vi "CRYO_MASTER_temp_0911.vi"() -> ()   [LabVIEW 2017] (continued)
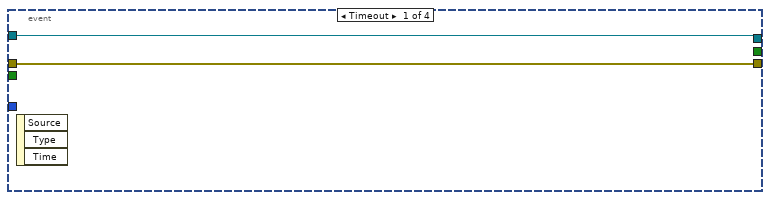
[diagram p3: hidden frame]
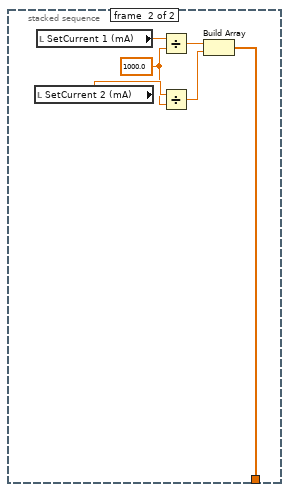
[diagram p8: hidden frame]
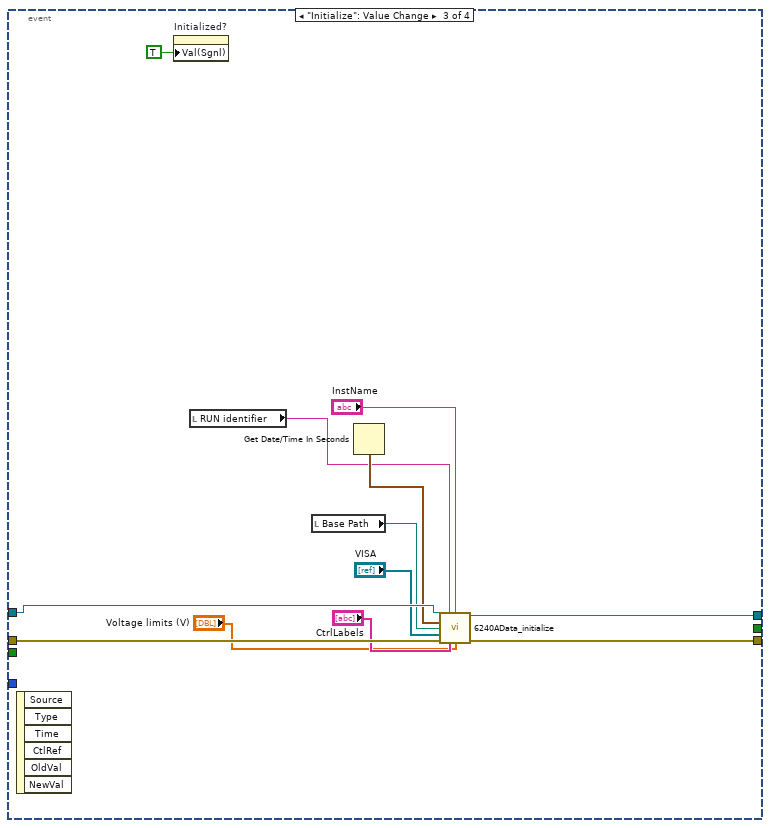
[diagram p10: hidden frame]
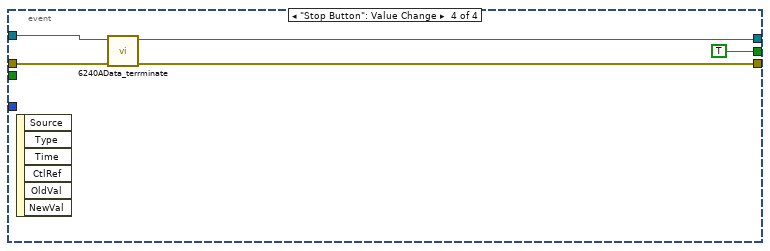
[diagram p11: hidden frame]
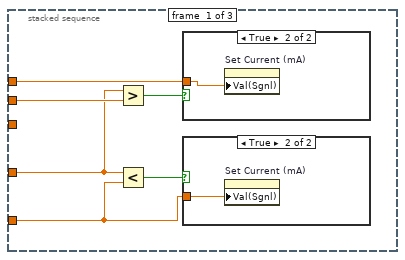
[diagram p12: hidden frame]
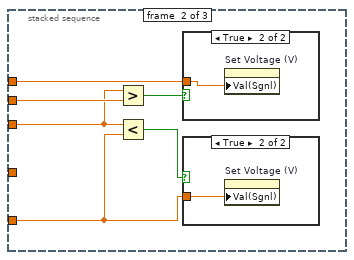
[diagram p15: hidden frame]
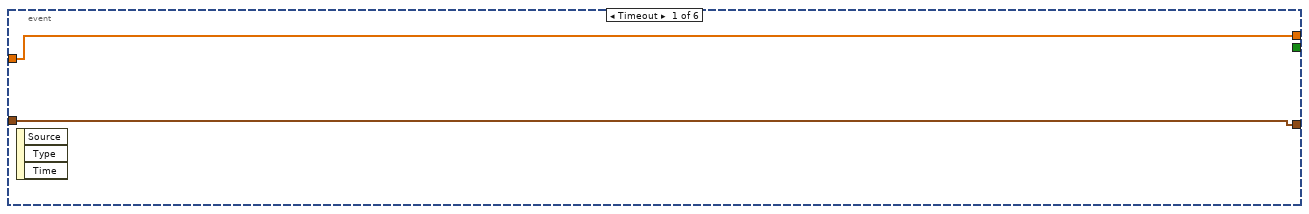
[diagram p18: hidden frame]
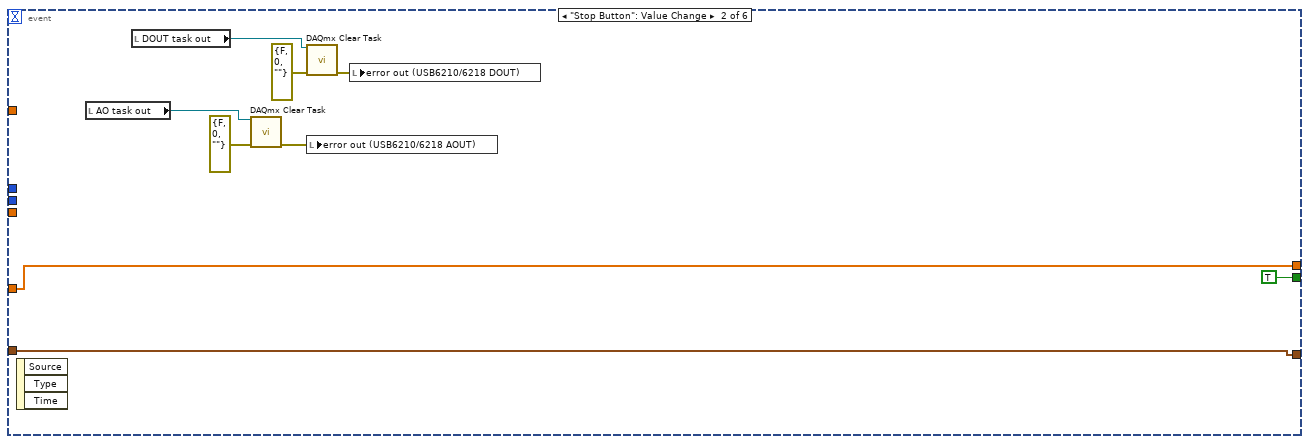
[diagram p19: hidden frame]
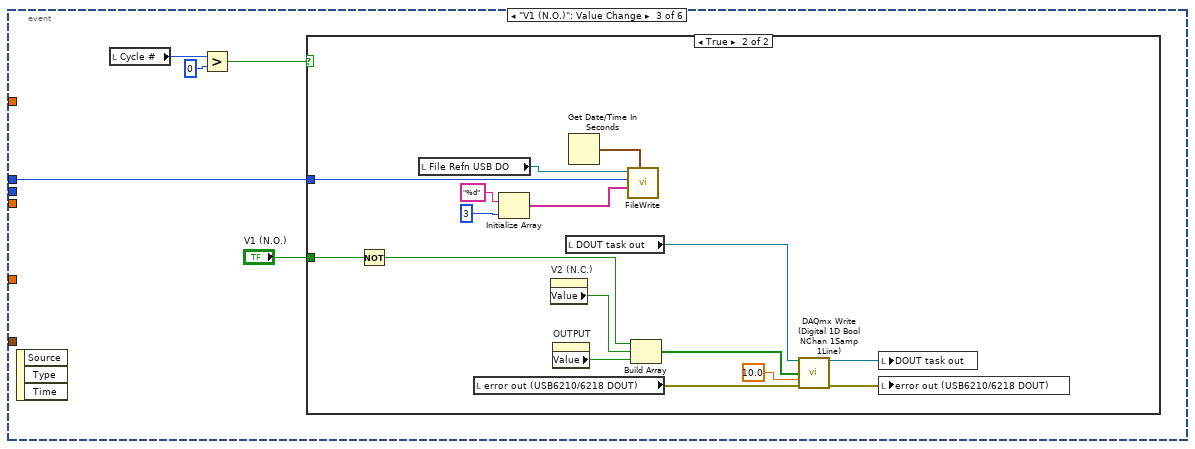
[diagram p20: hidden frame]
        "Time of Last Measurement (USB6218)" <- w698
        "Last Vol \n(USB6218)" <- w685
        n285 = call-dynamic "USBData_convert.vi"("Save every ... measurements"=w679, "MeasurementIndex"=w680, "error in (no error)"=w697, "LastDataAcquired"=w685, "TimeMeasuremeent"=w698, "USBData in"=w701) -> ("error out"=w696:errorcluster, "LeakDet_FULL"=w691:dbl, "LastDataConverted"=w686:dbl[], "USBData out"=w694:refnum<class "USBData.lvclass">)  [unwired: 2 in]
        n286 = call "USBData_read.vi"("USBData in"=w694, "error in (no error)"=w696) -> ("Status"=w687:T5, "USBData out"=w693:refnum<class "USBData.lvclass">, "Data"=w692:T15, "Basic"=w684:T16, "error out"=w695:errorcluster)  [unwired: 2 in, 2 out]
        n287 = local write "USB6218 Status"(w687) -> ()
        n288 = Unbundle By Name(w684) -> ("ReadLeakDet?"=w690:bool)
        n289 = Unbundle By Name(w684) -> ("Labels"=w683:string[])
        n290 = case shown="True" w690 {
          tunnel: w686 -> [w702 w705]
          tunnel: w691 -> [_ w704]
          tunnel: [w702 w703] -> w689
          frame False {
          }
          frame True {
            n291 = Build Array (concatenate)(w705, w704) -> (w703:dbl[])
          }
        }
        "Last Data \n(USB6218)" <- w689
      }
      frame True {
        n292 = Get Date/Time In Seconds() -> (seconds since 1Jan1904=w715:timestamp)
        n293 = call-dynamic "USBData_initialize.vi"("USBData in"=w711, "SeriesSetting"="USB6218 Config", "BasePath"=w710, "RunName"=w709, "FileName"="InstName (USB6218)", "error in (no error)"=w708, "RUN start time"=w715) -> ("Status"=w706:T5, "USBData out"=w724:refnum<class "USBData.lvclass">, "error out"=w725:errorcluster)  [unwired: 4 in, 2 out]
        n294 = local write "USB6218 Status"(w706) -> ()
        n295 = call "USBData_read.vi"("USBData in"=w724, "error in (no error)"=w725) -> ("Status"=w714:T5, "USBData out"=w721:refnum<class "USBData.lvclass">, "Data"=w722:T15, "Basic"=w716:T16, "error out"=w723:errorcluster)  [unwired: 2 in, 2 out]
        n296 = local write "USB6218 Status"(w714) -> ()
        n297 = Unbundle By Name(w716) -> ("ReadLeakDet?"=w720:bool, "Labels"=w713:string[])
        n298 = Array Size(array=w713) -> (size(s)=w719:i32)
        n299 = case shown="True" w720 {
          tunnel: w719 -> [w726 w728]
          tunnel: [w726 w727] -> w717
          frame False {
          }
          frame True {
            n300 = Add(x=w728, y=1) -> (x+y=w727:i32)
          }
        }
        n301 = Initialize Array(TRUE ("Activate 2"), w717) -> ()  [unwired: 1 out]
      }
    }
    "error out (USB6218)" <- w414
    n302 = case shown="False" w411 {
      tunnel: [w1080 w1095] -> w453
      tunnel: [w1075 w1094] -> w472
      tunnel: [w1078 w1093] -> w454
      tunnel: w422 -> [w1079 _]
      tunnel: w471 -> [w1069 w1088]
      tunnel: w470 -> [w1070 w1087]
      tunnel: w410 -> [_ w1086]
      tunnel: w409 -> [_ w1085]
      tunnel: [w1067 timestamp[] [] ("TimeArray")] -> w469
      tunnel: [w1066 dbl[][] [] ("DataArray")] -> w468
      frame False {
        w1073 = 24 ("index")
        n303 = local read "Record interval"() -> (w1064:i64)
        n304 = call-dynamic "LSI218Data_measure.vi"("LSI218Data in"=w1070, "MeasurementIndex"=w1079, "error in (no error)"=w1069, "save every ... measurements"=w1064) -> ("TimeMeasuremeent"=→"Time of Last Measurement (LSI218)":timestamp, "Active?"=w1074:bool[], "LSI218Data out"=w1078:refnum<class "LSI218Data.lvclass">, "LastMeasurementConfig"=→"LastMeasurementConfig (218)":T11, "LastData"=w1068:dbl[], "Status"=w1075:u16, "TimeArray"=w1067:timestamp[], "DataArray"=w1066:dbl[][], "error out"=w1080:errorcluster)  [unwired: 3 in]
        n305 = Split 1D Array(array=w1074, index=w1073) -> (first subarray=→"Active?\n (1)":bool[], second subarray=→"Active?\n(2)":bool[])
        n306 = Split 1D Array(array=w1068, index=w1073) -> (first subarray=→"Last Data \nLSI218 (1)":dbl[], second subarray=→"Last Data \nLSI218 (2)":dbl[])
      }
      frame True {
        n307 = Get Date/Time In Seconds() -> (seconds since 1Jan1904=w1096:timestamp)
        n308 = call-dynamic "LSI218Data_initialize.vi"("LSI218Settings(A-F)"="LSI218Settings(A-F)", "FileFormat"="FileFormat (218)", "RUN start time"=w1096, "base path"=w1085, "error in (no error)"=w1088, "InstName"="InstName (LSI218)", "RunName"=w1086, "LSI218Data in"=w1087) -> ("error out"=w1095:errorcluster, "Status"=w1094:T6, "AllLabels"=w1084:string[], "LSI218Data out"=w1093:refnum<class "LSI218Data.lvclass">)
        n309 = Split 1D Array(array=w1084, index=24) -> (first subarray=→"Labels LSI218 (1)":string[], second subarray=→"Labels LSI218 (2)":string[])
      }
    }
    "LSI218 Status" <- w472
    "error out (LSI218)" <- w453
    n310 = property on="Property Node" class="Arr (strict)"(reference=w431, "Number of Rows"=u32 8) -> ()  [unwired: 1 in, 2 out]
    n311 = Multiply(x="Measurement Interval (s)", y=u32 1000) -> (x*y=w474:dbl)
    n312 = Wait (ms)(milliseconds to wait=w474) -> ()  [unwired: 1 out]
    n313 = And(x="Analog Out ON?", y=w411) -> (x .and. y?=w412:bool)
    n314 = case shown="True" w412 {
      tunnel: w409 -> [_ w498]
      tunnel: w410 -> [_ w497]
      tunnel: [w483 w485] -> w408
      tunnel: w407 -> [w483 w484]
      frame False {
      }
      frame True {
        w496 = "_"
        w506 = 10.0 ("V_lim_max")
        w505 = 0.0 ("V_lim_min")
        w504 = -1 items=["Default"=-1, "RSE"=10083, "Differential"=10106, "Pseudodifferential"=12529] ("output terminal configuration")
        w503 = 10348 items=["Volts"=10348, "From Custom Scale"=10065] ("units")
        n315 = Get Date/Time In Seconds() -> (seconds since 1Jan1904=w501:timestamp)
        n316 = call "LV_UNIXTIME.vi"("current time"=w501) -> ("date/time string"=w494:string)  [unwired: 9 in, 1 out]
        n317 = Concatenate Strings(w497, w496, w494, w496, "USB_AOUT.csv" ("string")) -> (w499:string)
        n318 = Build Array("AOUT 0 Label", "AOUT 1 Label") -> (w487:string[])
        n319 = Build Path(base path=w498, name or relative path=w499) -> (appended path=w493:path)
        n320 = Concatenate Strings(w494, "_AO" ("string")) -> (w508:string)
        n321 = Open/Create/Replace File(file path (use dialog)=w493, operation (0:open)=T13."open or create") -> (refnum out=w491:refnum<file>)  [unwired: 4 in, 2 out]
        n322 = call "FileIntialize.vi"("Error In"=w484, "Labels"=w487, "refnum in"=w491) -> ("Error Out"=w486:errorcluster, "File Refnum"=→"File Refn USB AO":refnum<file>)  [unwired: 7 in]
        n323 = call <vilib>:"DAQmx Create Task.vi"("new task name"=w508, "auto cleanup"=FALSE, "error in"=w486) -> ("task out"=w507:refnum<k21>, "error out"=w509:errorcluster)  [unwired: 11 in]
        n324 = call-poly <vilib>:"DAQmx Create Virtual Channel.vi"("task in"=w507, "maximum value"=w506, "minimum value"=w505, "output terminal configuration"=w504, "physical channels"="AOUT For Voltage CTRL", "units"=w503, "error in"=w509) -> ("task out"=w511:refnum<k21>, "error out"=w512:errorcluster)  [unwired: 7 in]
        n325 = call-poly <vilib>:"DAQmx Create Virtual Channel.vi"("task in"=w511, "maximum value"=w506, "minimum value"=w505, "physical channels"="AOUT for Current CTRL", "error in"=w512) -> ("task out"=w514:refnum<k21>, "error out"=w513:errorcluster)  [unwired: 9 in]
        n326 = call <vilib>:"DAQmx Start Task.vi"("task/channels in"=w514, "error in"=w513) -> ("task out"=→"AO task out":refnum<k21>, "error out"=w485:errorcluster)  [unwired: 12 in]
      }
    }
    "error out (USB6210/6218 AOUT)" <- w408
    n327 = flat-sequence {
      tunnel: w478 -> [w613]
      tunnel: [w607] -> w465
      tunnel: [w605] -> w463
      tunnel: [w604] -> w460
      tunnel: [w603] -> w457
      tunnel: w425 -> [w598]
      frame #0 {
        w606 = T14 [] ("appended array")
        n328 = Unbundle By Name(w598) -> ("TimeArray"=w616:timestamp[], "DataArrayConv"=w611:dbl[][], "LDArray"=w610:dbl[])
        n329 = Unbundle By Name(w613) -> ("ReadLeakDet?"=w612:bool, "LabelLD"=w615:string, "Labels"=w608:string[])  [unwired: 1 out]
        n330 = case shown="True" w612 {
          tunnel: w615 -> [_ w624]
          tunnel: w611 -> [w618 w623]
          tunnel: w610 -> [_ w622]
          tunnel: [w618 w621] -> w609
          tunnel: w608 -> [w617 w620]
          tunnel: [w617 w619] -> w600
          frame False {
          }
          frame True {
            n331 = Build Array (concatenate)(w623, w622) -> (w621:dbl[][])
            n332 = Build Array (concatenate)(w620, w624) -> (w619:string[])
          }
        }
        "All Labels (USB6210)" <- w600
        "DataArrayConv (USB6210)" <- w609
        n333 = local read "Plot selecter (USB6210)\n    1      2     3     4"() -> (w602:bool[][])
        n334 = control-ref of="Plot selecter (USB6210)\n    1      2     3     4"() -> (w599:refnum<vi>)
        n335 = Array Size(array=w600) -> (size(s)=w614:i32)
        n336 = Array Size(array=w600) -> (size(s)=w601:i32)
        n337 = property on="Property Node" class="Arr (strict)"(reference=w599, "Number of Rows"=w601) -> ()  [unwired: 1 in, 2 out]
        n338 = for {
          N: w614 -> [_]
          tunnel: w609 -> [w645]
          tunnel: w616 -> [w646]
          shift-right: [w640] -> w605
          shift-left: w606 -> [w643]
          shift-right: [w638] -> w603
          shift-left: w606 -> [w641]
          shift-right: [w639] -> w607
          shift-left: w606 -> [w637]
          shift-right: [w636] -> w604
          shift-left: w606 -> [w635]
          tunnel: w602 -> [w634]
          i -> [w629]
          n339 = Index Array(array=w645, index (col)=w629) -> (element=w644:dbl[])  [unwired: 1 in]
          n340 = Index Array(array=w634, index (row) #1=w629, index (col) #1=0 ("index (row)"), index (row) #2=w629, index (col) #2=1 ("index (row)"), index (row) #3=w629, index (col) #3=2 ("index (row)"), index (row) #4=w629, index (col) #4=3 ("index (row)")) -> (element #1=w628:bool, element #2=w627:bool, element #3=w626:bool, element #4=w625:bool)
          n341 = Bundle("TimeArray"=w646, "DataArrayConv"=w644) -> (w642:T17)  [unwired: 1 in]
          n342 = stacked-sequence {
            tunnel: w628 -> [w650 _ _ _]
            tunnel: w643 -> [_ w658 _ _]
            tunnel: w626 -> [_ _ w666 _]
            tunnel: w642 -> [w647 w656 w665 w671]
            tunnel: w625 -> [_ _ _ w674]
            tunnel: w641 -> [_ _ _ w673]
            tunnel: [_ _ _ w672] -> w638
            tunnel: [_ w657 _ _] -> w640
            tunnel: [w649 _ _ _] -> w639
            tunnel: w637 -> [w648 _ _ _]
            tunnel: [_ _ w664 _] -> w636
            tunnel: w635 -> [_ _ w663 _]
            tunnel: w627 -> [_ w655 _ _]
            frame #0 {
              n343 = case shown="True" w650 {
                tunnel: [w651 w654] -> w649
                tunnel: w647 -> [_ w653]
                tunnel: w648 -> [w651 w652]
                frame False {
                }
                frame True {
                  n344 = Build Array (concatenate)(w652, w653) -> (w654:T14)
                }
              }
            }
            frame #1 {
              n345 = case shown="True" w655 {
                tunnel: w658 -> [w659 w662]
                tunnel: [w659 w661] -> w657
                tunnel: w656 -> [_ w660]
                frame False {
                }
                frame True {
                  n346 = Build Array (concatenate)(w662, w660) -> (w661:T14)
                }
              }
            }
            frame #2 {
              n347 = case shown="True" w666 {
                tunnel: [w667 w670] -> w664
                tunnel: w665 -> [_ w669]
                tunnel: w663 -> [w667 w668]
                frame False {
                }
                frame True {
                  n348 = Build Array (concatenate)(w668, w669) -> (w670:T14)
                }
              }
            }
            frame #3 {
              n349 = case shown="True" w674 {
                tunnel: [w675 w678] -> w672
                tunnel: w671 -> [_ w677]
                tunnel: w673 -> [w675 w676]
                frame False {
                }
                frame True {
                  n350 = Build Array (concatenate)(w676, w677) -> (w678:T14)
                }
              }
            }
          }
        }
      }
    }
    n351 = flat-sequence {
      tunnel: w420 -> [w532]
      tunnel: [w526] -> w419
      tunnel: [w524] -> w418
      tunnel: [w523] -> w417
      tunnel: [w522] -> w416
      tunnel: w421 -> [w518]
      frame #0 {
        w525 = T14 [] ("appended array")
        n352 = Unbundle By Name(w518) -> ("TimeArray"=w535:timestamp[], "DataArrayConv"=w530:dbl[][], "LDArray"=w529:dbl[])
        "TimeArray (USB6218)" <- w535
        n353 = Unbundle By Name(w532) -> ("ReadLeakDet?"=w531:bool, "LabelLD"=w534:string, "Labels"=w527:string[])  [unwired: 1 out]
        n354 = case shown="True" w531 {
          tunnel: w534 -> [_ w543]
          tunnel: w530 -> [w537 w542]
          tunnel: w529 -> [_ w541]
          tunnel: [w537 w540] -> w528
          tunnel: w527 -> [w536 w539]
          tunnel: [w536 w538] -> w519
          frame False {
          }
          frame True {
            n355 = Build Array (concatenate)(w542, w541) -> (w540:dbl[][])
            n356 = Build Array (concatenate)(w539, w543) -> (w538:string[])
          }
        }
        "All Labels (USB6218)" <- w519
        "DataArrayConv (USB6218)" <- w528
        n357 = control-ref of="Plot selecter (USB6218)\n    1      2     3     4"() -> (w517:refnum<vi>)
        n358 = local read "Plot selecter (USB6218)\n    1      2     3     4"() -> (w521:bool[][])
        n359 = Array Size(array=w519) -> (size(s)=w533:i32)
        n360 = Array Size(array=w519) -> (size(s)=w520:i32)
        n361 = property on="Property Node" class="Arr (strict)"(reference=w517, "Number of Rows"=w520) -> ()  [unwired: 1 in, 2 out]
        n362 = for {
          N: w533 -> [_]
          tunnel: w528 -> [w564]
          tunnel: w535 -> [w565]
          shift-right: [w559] -> w524
          shift-left: w525 -> [w562]
          shift-right: [w557] -> w522
          shift-left: w525 -> [w560]
          shift-right: [w558] -> w526
          shift-left: w525 -> [w556]
          shift-right: [w555] -> w523
          shift-left: w525 -> [w554]
          tunnel: w521 -> [w553]
          i -> [w548]
          n363 = Index Array(array=w564, index (col)=w548) -> (element=w563:dbl[])  [unwired: 1 in]
          n364 = Index Array(array=w553, index (row) #1=w548, index (col) #1=0 ("index (row)"), index (row) #2=w548, index (col) #2=1 ("index (row)"), index (row) #3=w548, index (col) #3=2 ("index (row)"), index (row) #4=w548, index (col) #4=3 ("index (row)")) -> (element #1=w547:bool, element #2=w546:bool, element #3=w545:bool, element #4=w544:bool)
          n365 = Bundle("TimeArray"=w565, "DataArrayConv"=w563) -> (w561:T17)  [unwired: 1 in]
          n366 = stacked-sequence {
            tunnel: w547 -> [w569 _ _ _]
            tunnel: w562 -> [_ w577 _ _]
            tunnel: w545 -> [_ _ w585 _]
            tunnel: w561 -> [w566 w575 w584 w590]
            tunnel: w544 -> [_ _ _ w593]
            tunnel: w560 -> [_ _ _ w592]
            tunnel: [_ _ _ w591] -> w557
            tunnel: [_ w576 _ _] -> w559
            tunnel: [w568 _ _ _] -> w558
            tunnel: w556 -> [w567 _ _ _]
            tunnel: [_ _ w583 _] -> w555
            tunnel: w554 -> [_ _ w582 _]
            tunnel: w546 -> [_ w574 _ _]
            frame #0 {
              n367 = case shown="True" w569 {
                tunnel: [w570 w573] -> w568
                tunnel: w566 -> [_ w572]
                tunnel: w567 -> [w570 w571]
                frame False {
                }
                frame True {
                  n368 = Build Array (concatenate)(w571, w572) -> (w573:T14)
                }
              }
            }
            frame #1 {
              n369 = case shown="True" w574 {
                tunnel: w577 -> [w578 w581]
                tunnel: [w578 w580] -> w576
                tunnel: w575 -> [_ w579]
                frame False {
                }
                frame True {
                  n370 = Build Array (concatenate)(w581, w579) -> (w580:T14)
                }
              }
            }
            frame #2 {
              n371 = case shown="True" w585 {
                tunnel: [w586 w589] -> w583
                tunnel: w584 -> [_ w588]
                tunnel: w582 -> [w586 w587]
                frame False {
                }
                frame True {
                  n372 = Build Array (concatenate)(w587, w588) -> (w589:T14)
                }
              }
            }
            frame #3 {
              n373 = case shown="True" w593 {
                tunnel: [w594 w597] -> w591
                tunnel: w590 -> [_ w596]
                tunnel: w592 -> [w594 w595]
                frame False {
                }
                frame True {
                  n374 = Build Array (concatenate)(w595, w596) -> (w597:T14)
                }
              }
            }
          }
        }
      }
    }
    n375 = local read "Plot selecter LSI218(1)\n    1      2     3     4"() -> (w452:bool[][])
    n376 = local read "Plot selecter LSI218(2)\n    1      2     3     4"() -> (w451:bool[][])
    n377 = for {
      N: 48 -> [_]
      tunnel: w469 -> [w1008]
      tunnel: w468 -> [w1005]
      tunnel: w452 -> [w989]
      tunnel: w451 -> [w990]
      shift-right: [w1006] -> w467
      shift-left: w464 -> [w1007]
      shift-right: [w1001] -> w461
      shift-left: w464 -> [w1002]
      shift-right: [w1000] -> w458
      shift-left: w464 -> [w999]
      shift-right: [w998] -> w456
      shift-left: w464 -> [w997]
      i -> [w995]
      n378 = Index Array(array=w1005, index (col)=w995) -> (element=w1004:dbl[])  [unwired: 1 in]
      n379 = Less?(x=w995, y=24) -> (x < y?=w996:bool)
      n380 = case shown="True" w996 {
        tunnel: [w1013 w1031] -> w994
        tunnel: [w1012 w1030] -> w993
        tunnel: [w1011 w1028] -> w992
        tunnel: [w1010 w1027] -> w991
        tunnel: w989 -> [_ w1026]
        tunnel: w990 -> [w1020 _]
        tunnel: w995 -> [w1015 w1023]
        frame False {
          n381 = Subtract(x=w1015, y=24) -> (x-y=w1019:i32)
          n382 = Index Array(array=w1020, index (row) #1=w1019, index (col) #1=0 ("index (row)"), index (row) #2=w1019, index (col) #2=1 ("index (row)"), index (row) #3=w1019, index (col) #3=2 ("index (row)"), index (row) #4=w1019, index (col) #4=3 ("index (row)")) -> (element #1=w1013:bool, element #2=w1012:bool, element #3=w1011:bool, element #4=w1010:bool)
        }
        frame True {
          n383 = Index Array(array=w1026, index (row) #1=w1023, index (col) #1=0 ("index (row)"), index (row) #2=w1023, index (col) #2=1 ("index (row)"), index (row) #3=w1023, index (col) #3=2 ("index (row)"), index (row) #4=w1023, index (col) #4=3 ("index (row)")) -> (element #1=w1031:bool, element #2=w1030:bool, element #3=w1028:bool, element #4=w1027:bool)
        }
      }
      n384 = Bundle("TimeArray"=w1008, "DataArray"=w1004) -> (w1003:T18)  [unwired: 1 in]
      n385 = stacked-sequence {
        tunnel: w1007 -> [w1035 _ _ _]
        tunnel: [w1034 _ _ _] -> w1006
        tunnel: w1003 -> [w1033 w1043 w1051 w1059]
        tunnel: w1002 -> [_ w1042 _ _]
        tunnel: [_ w1041 _ _] -> w1001
        tunnel: [_ _ w1050 _] -> w1000
        tunnel: w999 -> [_ _ w1049 _]
        tunnel: [_ _ _ w1058] -> w998
        tunnel: w997 -> [_ _ _ w1057]
        tunnel: w994 -> [w1032 _ _ _]
        tunnel: w993 -> [_ w1040 _ _]
        tunnel: w992 -> [_ _ w1048 _]
        tunnel: w991 -> [_ _ _ w1056]
        frame #0 {
          n386 = case shown="False" w1032 {
            tunnel: w1033 -> [_ w1037]
            tunnel: w1035 -> [w1036 w1039]
            tunnel: [w1036 w1038] -> w1034
            frame False {
            }
            frame True {
              n387 = Build Array (concatenate)(w1039, w1037) -> (w1038:T8)
            }
          }
        }
        frame #1 {
          n388 = case shown="True" w1040 {
            tunnel: [w1044 w1047] -> w1041
            tunnel: w1043 -> [_ w1046]
            tunnel: w1042 -> [w1044 w1045]
            frame False {
            }
            frame True {
              n389 = Build Array (concatenate)(w1045, w1046) -> (w1047:T8)
            }
          }
        }
        frame #2 {
          n390 = case shown="True" w1048 {
            tunnel: [w1052 w1055] -> w1050
            tunnel: w1051 -> [_ w1054]
            tunnel: w1049 -> [w1052 w1053]
            frame False {
            }
            frame True {
              n391 = Build Array (concatenate)(w1053, w1054) -> (w1055:T8)
            }
          }
        }
        frame #3 {
          n392 = case shown="True" w1056 {
            tunnel: [w1060 w1063] -> w1058
            tunnel: w1059 -> [_ w1062]
            tunnel: w1057 -> [w1060 w1061]
            frame False {
            }
            frame True {
              n393 = Build Array (concatenate)(w1061, w1062) -> (w1063:T8)
            }
          }
        }
      }
    }
    n394 = local read "Plot selecter LSI336 \n     1      2     3     4"() -> (w447:bool[][])
    n395 = local read "Labels LSI336"() -> (w437:string[])
    n396 = Array Size(array=w437) -> (size(s)=w436:i32)
    n397 = case shown="True" "Digital Out ON?" {
      tunnel: w411 -> [_ w737]
      tunnel: w428 -> [_ w736]
      tunnel: w427 -> [w730 w735]
      tunnel: [w730 w734] -> w426
      tunnel: w425 -> [_ w733]
      tunnel: w410 -> [_ w732]
      tunnel: w409 -> [_ w731]
      frame False {
      }
      frame True {
        n398 = case shown="True" w737 {
          tunnel: w736 -> [_ w907]
          tunnel: w735 -> [w747 w866]
          tunnel: [w747 w888] -> w734
          tunnel: w733 -> [w748 _]
          tunnel: w732 -> [_ w876]
          tunnel: w731 -> [_ w858]
          frame False {
            n399 = Multiply(x="N for sampling", y=i64 2) -> (x*y=w742:i64)
            n400 = local read "Cycle #"() -> (w746:u32)
            n401 = Add(x=w742, y="Mov. Avg Interval") -> (x+y=w744:i64)
            n402 = Greater?(x=w746, y=w744) -> (0:w740:bool)
            n403 = And(x=w740, y="Auto ON?") -> (x .and. y?=w738:bool)
            n404 = case shown="True" w738 {
              tunnel: w748 -> [_ w770]
              tunnel: "Mov. Avg Interval" -> [_ w752]
              tunnel: w742 -> [_ w754]
              tunnel: "N for sampling" -> [_ w749]
              frame False {
              }
              frame True {
                # "Need to record the valve status"
                n405 = Unbundle By Name(w770) -> ("TimeArray"=w768:timestamp[], "DataArrayConv"=w769:dbl[][])
                n406 = Reciprocal(x=w752) -> (1/x=w767:dbl)
                n407 = local read "Pstd"() -> (→"Pstd history":dbl)
                n408 = local read "Pav"() -> (→"Pav history":dbl)
                n409 = local read "Target Index"() -> (w771:i32)
                n410 = Index Array(array=w769, index (col)=w771) -> (element=w762:dbl[])  [unwired: 1 in]
                n411 = Initialize Array(w767, w752) -> (w766:dbl[])
                n412 = Delete From Array(array=w762, length=w754) -> (deleted portion=w761:dbl[])  [unwired: 1 in, 1 out]
                n413 = call-poly <vilib>:"FIR Filter.vi"("FIR Coefficients"=w766, "X"=w762) -> ("Filtered X"=w759:dbl[])  [unwired: 2 in, 1 out]
                n414 = Delete From Array(array=w768, length=w754) -> (deleted portion=w765:timestamp[])  [unwired: 1 in, 1 out]
                n415 = Delete From Array(array=w759, length=w754) -> (deleted portion=w763:dbl[])  [unwired: 1 in, 1 out]
                n416 = Delete From Array(array=w759, length=w749) -> (deleted portion=w757:dbl[])  [unwired: 1 in, 1 out]
                "Last N M.A. Pressures" <- w757
                n417 = Bundle("TimeArray"=w765, "DataArrayConv"=w761) -> (w760:T17)  [unwired: 1 in]
                n418 = Bundle("TimeArray"=w765, "Filtered X"=w763) -> (w764:T19)  [unwired: 1 in]
                n419 = Build Array(w760, w764) -> (→"Graph 5":T9)
                n420 = Array Size(array=w757) -> (size(s)=w756:i32)
                n421 = Equal?(x=w756, y=w749) -> (x = y?=w755:bool)
                n422 = case shown="True" w755 {
                  tunnel: [nan ("mean") w774] -> w753
                  tunnel: w757 -> [_ w775]
                  frame False {
                  }
                  frame True {
                    n423 = call <vilib>:"Std Deviation and Variance.vi"("X"=w775) -> ("mean"=w774:dbl, "standard deviation"=w773:dbl)  [unwired: 1 in, 1 out]
                    n424 = local write "Pav"(w774) -> ()
                    n425 = local write "Pstd"(w773) -> ()
                  }
                }
                n426 = stacked-sequence {
                  tunnel: w753 -> [w778 w790 w802 w814 w827 _]
                  frame #0 {
                    n427 = local read "P_1_th_high (Pa)"() -> (w785:dbl)
                    n428 = local read "P_1_tol (Pa)"() -> (w786:dbl)
                    n429 = local read "V1 (N.O.)"() -> (w783:bool)
                    n430 = local write "Status V1 CTRL"(enum16{"Pressurize", "Depressurize"}."Depressurize" ("Status V1 CTRL")) -> ()
                    n431 = Add(x=w785, y=w786) -> (x+y=w777:dbl)
                    n432 = Subtract(x=w778, y=w777) -> (x-y=→"Pav - (P_1_th_high+P_1_tol)=":dbl)
                    n433 = Greater?(x=w778, y=w777) -> (0:w784:bool)
                    n434 = Equal?(x=w783, y=FALSE) -> (x = y?=w781:bool)
                    n435 = And(x=w784, y=w781) -> (x .and. y?=w780:bool)
                    n436 = case shown="True" w780 {
                      frame False {
                      }
                      frame True {
                        n437 = property on="V1 (N.O.)" class="Bool (strict)"("Val(Sgnl)"=TRUE ("V1 (N.O.)")) -> ()  [unwired: 2 in, 2 out]
                      }
                    }
                  }
                  frame #1 {
                    n438 = local read "P_2_th_high (Pa)"() -> (w797:dbl)
                    n439 = local read "P_2_tol (Pa)"() -> (w798:dbl)
                    n440 = local read "V2 (N.C.)"() -> (w795:bool)
                    n441 = local write "Status V2 CTRL"(enum16{"Pressurize", "Depressurize"}."Depressurize" ("Status V2 CTRL")) -> ()
                    n442 = Add(x=w797, y=w798) -> (x+y=w789:dbl)
                    n443 = Subtract(x=w790, y=w789) -> (x-y=→"Pav - (P_2_th_high+P_2_tol)=":dbl)
                    n444 = Greater?(x=w790, y=w789) -> (0:w796:bool)
                    n445 = Equal?(x=w795, y=TRUE) -> (x = y?=w793:bool)
                    n446 = And(x=w796, y=w793) -> (x .and. y?=w792:bool)
                    n447 = case shown="True" w792 {
                      frame False {
                      }
                      frame True {
                        n448 = property on="V2 (N.C.)" class="Bool (strict)"("Val(Sgnl)"=FALSE ("V1 (N.O.)")) -> ()  [unwired: 2 in, 2 out]
                      }
                    }
                  }
                  frame #2 {
                    n449 = local read "P_1_th_low (Pa)"() -> (w809:dbl)
                    n450 = local read "P_1_tol (Pa)"() -> (w810:dbl)
                    n451 = local write "Status V1 CTRL"(enum16{"Pressurize", "Depressurize"}."Pressurize" ("Status V1 CTRL")) -> ()
                    n452 = local read "V1 (N.O.)"() -> (w807:bool)
                    n453 = Subtract(x=w809, y=w810) -> (x-y=w801:dbl)
                    n454 = Subtract(x=w802, y=w801) -> (x-y=→"Pav - (P_1_th_low_-P_1_tol)=":dbl)
                    n455 = Less?(x=w802, y=w801) -> (x < y?=w808:bool)
                    n456 = Equal?(x=w807, y=TRUE) -> (x = y?=w805:bool)
                    n457 = And(x=w808, y=w805) -> (x .and. y?=w804:bool)
                    n458 = case shown="True" w804 {
                      frame False {
                      }
                      frame True {
                        n459 = property on="V1 (N.O.)" class="Bool (strict)"("Val(Sgnl)"=FALSE ("V1 (N.O.)")) -> ()  [unwired: 2 in, 2 out]
                      }
                    }
                  }
                  frame #3 {
                    n460 = local read "P_2_th_low (Pa)"() -> (w821:dbl)
                    n461 = local read "P_2_tol (Pa)"() -> (w822:dbl)
                    n462 = local write "Status V2 CTRL"(enum16{"Pressurize", "Depressurize"}."Pressurize" ("Status V2 CTRL")) -> ()
                    n463 = local read "V2 (N.C.)"() -> (w819:bool)
                    n464 = Subtract(x=w821, y=w822) -> (x-y=w813:dbl)
                    n465 = Subtract(x=w814, y=w813) -> (x-y=→"Pav - (P_2_th_low_-P_2_tol)=":dbl)
                    n466 = Less?(x=w814, y=w813) -> (x < y?=w820:bool)
                    n467 = Equal?(x=w819, y=FALSE) -> (x = y?=w817:bool)
                    n468 = And(x=w820, y=w817) -> (x .and. y?=w816:bool)
                    n469 = case shown="True" w816 {
                      frame False {
                      }
                      frame True {
                        n470 = property on="V2 (N.C.)" class="Bool (strict)"("Val(Sgnl)"=TRUE ("V1 (N.O.)")) -> ()  [unwired: 2 in, 2 out]
                      }
                    }
                  }
                  frame #4 {
                    n471 = Greater?(x=w827, y="P_safelimit_up (Pa)") -> (0:w828:bool)
                    n472 = Less?(x=w827, y="P_safelimit_low (Pa)") -> (x < y?=w825:bool)
                    n473 = Or(x=w828, y=w825) -> (x .or. y?=w824:bool)
                    n474 = case shown="True" w824 {
                      frame False {
                      }
                      frame True {
                        n475 = property on="V2 (N.C.)" class="Bool (strict)"("Val(Sgnl)"=FALSE ("V1 (N.O.)")) -> ()  [unwired: 2 in, 2 out]
                        n476 = property on="V1 (N.O.)" class="Bool (strict)"("Val(Sgnl)"=TRUE ("V1 (N.O.)")) -> ()  [unwired: 2 in, 2 out]
                      }
                    }
                  }
                  frame #5 {
                    n477 = local read "P_1_th_high (Pa)"() -> (w842:dbl)
                    n478 = local read "P_2_th_high (Pa)"() -> (w839:dbl)
                    n479 = local read "P_1_th_low (Pa)"() -> (w843:dbl)
                    n480 = local read "P_2_th_low (Pa)"() -> (w840:dbl)
                    n481 = property on="V1 (N.O.)" class="Bool (strict)"() -> ("Value"=w835:bool)  [unwired: 2 in, 2 out]
                    n482 = property on="V2 (N.C.)" class="Bool (strict)"() -> ("Value"=w837:bool)  [unwired: 2 in, 2 out]
                    n483 = local read "P_1_tol (Pa)"() -> (w841:dbl)
                    n484 = local read "P_2_tol (Pa)"() -> (w838:dbl)
                    n485 = Boolean To (0,1)(Boolean=w835) -> (0, 1=w834:i16)
                    n486 = Boolean To (0,1)(Boolean=w837) -> (0, 1=w836:i16)
                    n487 = local read "File Refn DewarCTRL"() -> (w844:refnum<file>)
                    n488 = local read "Pav"() -> (w850:dbl)
                    n489 = local read "Cycle #"() -> (w849:u32)
                    n490 = Build Array(w850, w843, w842, w841, w840, w839, w838, w834, w836) -> (w833:dbl[])
                    n491 = Get Date/Time In Seconds() -> (seconds since 1Jan1904=w845:timestamp)
                    n492 = call "FileWrite.vi"("DataArray"=w833, "Time Stamp"=w845, "Error In"=errorcluster {"status"=FALSE, "code"=0, "source"=""}, "FileFormat"=string[] ["%4.5e", "%4.4e", "%4.4e", "%4.4e", "%4.4e", "%4.4e", "%4.4e", "%d", "%d"] ("Array"), "Index"=w849, "refnum in"=w844) -> ("Error Out"=→"Error Out (Dewar CTRL":errorcluster, "Byte Stream File Refnum"=w832:refnum<file>)  [unwired: 4 in]
                    n493 = local write "File Refn DewarCTRL"(w832) -> ()
                  }
                }
              }
            }
          }
          frame True {
            (unwired) "_"
            w882 = "_"
            w868 = FALSE ("auto cleanup")
            w887 = 1 items=["one channel for each line", "one channel for all lines"] ("line grouping")
            n494 = Get Date/Time In Seconds() -> (seconds since 1Jan1904=w903:timestamp)
            n495 = local write "V2 (N.C.)"(FALSE ("V1 (N.O.)")) -> ()
            n496 = local write "V1 (N.O.)"(TRUE ("V1 (N.O.)")) -> ()
            n497 = call "LV_UNIXTIME.vi"("current time"=w903) -> ("date/time string"=w877:string)  [unwired: 9 in, 1 out]
            n498 = Search 1D Array(1D array=w907, element="Dewar Regularization \nTarget Signal Label") -> (index of element=→"Target Index":i32)  [unwired: 1 in]
            n499 = Concatenate Strings(w877, "_DO" ("new task name")) -> (w900:string)
            n500 = Concatenate Strings(w876, w882, w877, w882) -> (w857:string)
            n501 = Concatenate Strings(w857, "DEWARcsv" ("string")) -> (w856:string)
            n502 = Concatenate Strings(w857, "USB_DOUT.csv" ("string")) -> (w860:string)
            n503 = Build Path(base path=w858, name or relative path=w856) -> (appended path=w855:path)
            n504 = Build Path(base path=w858, name or relative path=w860) -> (appended path=w881:path)
            n505 = Open/Create/Replace File(file path (use dialog)=w881, error in=w866, operation (0:open)=T13."open or create") -> (refnum out=w879:refnum<file>, error out=w865:errorcluster)  [unwired: 3 in, 1 out]
            n506 = call "FileIntialize.vi"("Error In"=w865, "Labels"="DOUT Labels", "refnum in"=w879) -> ("Error Out"=w852:errorcluster, "File Refnum"=→"File Refn USB DO":refnum<file>)  [unwired: 7 in]
            n507 = Open/Create/Replace File(file path (use dialog)=w855, error in=w852, operation (0:open)=T13."open or create") -> (refnum out=w863:refnum<file>, error out=w864:errorcluster)  [unwired: 3 in, 1 out]
            n508 = call "FileIntialize.vi"("Error In"=w864, "Labels"=string[] ["P_av", "P_1_th_high", "P_1_th_low", "P_1_tol", "P_2_th_high", "P_2_th_low", "P_2_tol", "V1", "V2"], "refnum in"=w863) -> ("Error Out"=w851:errorcluster, "File Refnum"=→"File Refn DewarCTRL":refnum<file>)  [unwired: 7 in]
            n509 = Index Array(array="DOUT Physical CH", index=2) -> (element=w869:tag)
            n510 = Index Array(array="DOUT Physical CH", index=1) -> (element=w872:tag)
            n511 = Index Array(array="DOUT Physical CH", index=0) -> (element=w874:tag)
            n512 = call <vilib>:"DAQmx Create Task.vi"("new task name"=w900, "auto cleanup"=FALSE, "error in"=w851) -> ("task out"=w901:refnum<k21>, "error out"=w902:errorcluster)  [unwired: 11 in]
            n513 = call-poly <vilib>:"DAQmx Create Virtual Channel.vi"("task in"=w901, "lines"=w874, "line grouping"=w887, "error in"=w902) -> ("task out"=w904:refnum<k21>, "error out"=w905:errorcluster)  [unwired: 10 in]
            n514 = call-poly <vilib>:"DAQmx Create Virtual Channel.vi"("task in"=w904, "lines"=w872, "line grouping"=w887, "error in"=w905) -> ("task out"=w886:refnum<k21>, "error out"=w884:errorcluster)  [unwired: 10 in]
            n515 = call-poly <vilib>:"DAQmx Create Virtual Channel.vi"("task in"=w886, "lines"=w869, "line grouping"=w887, "error in"=w884) -> ("task out"=w885:refnum<k21>, "error out"=w883:errorcluster)  [unwired: 10 in]
            n516 = call <vilib>:"DAQmx Start Task.vi"("task/channels in"=w885, "error in"=w883) -> ("task out"=w891:refnum<k21>, "error out"=w889:errorcluster)  [unwired: 12 in]
            n517 = Build Array(FALSE ("auto cleanup"), w868, w868) -> (w892:bool[])
            n518 = call <vilib>:"DAQmx Write (Digital 1D Bool NChan 1Samp 1Line).vi"("task/channels in"=w891, "data"=w892, "timeout"=10.0, "error in"=w889) -> ("task out"=→"DOUT task out":refnum<k21>, "error out"=w888:errorcluster)  [unwired: 9 in, 1 out]
          }
        }
      }
    }
    "error out (USB6210/6218 DOUT)" <- w426
    n519 = for {
      N: w436 -> [_]
      tunnel: w447 -> [w920]
      shift-right: [w914] -> w443
      shift-left: w446 -> [w929]
      shift-right: [w910] -> w442
      shift-left: w446 -> [w927]
      shift-right: [w911] -> w441
      shift-left: w446 -> [w926]
      shift-right: [w909] -> w440
      shift-left: w446 -> [w925]
      tunnel: w445 -> [w917]
      tunnel: w444 -> [w915]
      i -> [w918]
      n520 = Index Array(array=w917, index (col)=w918) -> (element=w916:dbl[])  [unwired: 1 in]
      n521 = Index Array(array=w920, index (row) #1=w918, index (col) #1=0 ("index (row)"), index (row) #2=w918, index (col) #2=1 ("index (row)"), index (row) #3=w918, index (col) #3=2 ("index (row)"), index (row) #4=w918, index (col) #4=3 ("index (row)")) -> (element #1=w919:bool, element #2=w913:bool, element #3=w912:bool, element #4=w908:bool)
      n522 = Bundle("TimeArray"=w915, "DataArray"=w916) -> (w928:T18)  [unwired: 1 in]
      n523 = stacked-sequence {
        tunnel: w929 -> [w933 _ _ _]
        tunnel: [w932 _ _ _] -> w914
        tunnel: w928 -> [w931 w941 w949 w957]
        tunnel: w927 -> [_ w940 _ _]
        tunnel: [_ w939 _ _] -> w910
        tunnel: [_ _ w948 _] -> w911
        tunnel: w926 -> [_ _ w947 _]
        tunnel: [_ _ _ w956] -> w909
        tunnel: w925 -> [_ _ _ w955]
        tunnel: w919 -> [w930 _ _ _]
        tunnel: w913 -> [_ w938 _ _]
        tunnel: w912 -> [_ _ w946 _]
        tunnel: w908 -> [_ _ _ w954]
        frame #0 {
          n524 = case shown="False" w930 {
            tunnel: w931 -> [_ w935]
            tunnel: w933 -> [w934 w937]
            tunnel: [w934 w936] -> w932
            frame False {
            }
            frame True {
              n525 = Build Array (concatenate)(w937, w935) -> (w936:T8)
            }
          }
        }
        frame #1 {
          n526 = case shown="True" w938 {
            tunnel: [w942 w945] -> w939
            tunnel: w941 -> [_ w943]
            tunnel: w940 -> [w942 w944]
            frame False {
            }
            frame True {
              n527 = Build Array (concatenate)(w944, w943) -> (w945:T8)
            }
          }
        }
        frame #2 {
          n528 = case shown="False" w946 {
            tunnel: [w950 w953] -> w948
            tunnel: w949 -> [_ w951]
            tunnel: w947 -> [w950 w952]
            frame False {
            }
            frame True {
              n529 = Build Array (concatenate)(w952, w951) -> (w953:T8)
            }
          }
        }
        frame #3 {
          n530 = case shown="True" w954 {
            tunnel: [w958 w961] -> w956
            tunnel: w957 -> [_ w959]
            tunnel: w955 -> [w958 w960]
            frame False {
            }
            frame True {
              n531 = Build Array (concatenate)(w960, w959) -> (w961:T8)
            }
          }
        }
      }
    }
    n532 = Build Array (concatenate)(w465, w467, w443, w419) -> (→"Graph 1":T14)
    n533 = Build Array (concatenate)(w463, w461, w442, w418) -> (→"Graph 2":T14)
    n534 = Build Array (concatenate)(w457, w456, w440, w416) -> (→"Graph 4":T14)
    n535 = Build Array (concatenate)(w460, w458, w441, w417) -> (→"Graph 3":T14)
    "Cycle #" <- w422
  }
  n536 = while {
    shift-right: [w1159] -> _
    shift-left: refnum<class "6240AData.lvclass"> refnum ("6240AData.lvclass") -> [w1156]
    shift-right: [w1154] -> _
    shift-left: errorcluster {"status"=FALSE, "code"=0, "source"=""} ("error in (no error)") -> [w1155]
    i -> [w1153]
    stop <- w1157 stop-if-true
    n537 = Wait (ms)(milliseconds to wait=u32 231) -> ()  [unwired: 1 out]
    n538 = Equal?(x=w1153, y=0) -> (x = y?=w1151:bool)
    n539 = case shown="True" w1151 {
      frame False {
      }
      frame True {
        n540 = property on="Initialized?" class="Bool (strict)"("Val(Sgnl)"=FALSE ("Value (Signaling)")) -> ()  [unwired: 2 in, 2 out]
      }
    }
    n541 = event shown="[1] \"Output\", \"SetCurrent 1 (mA)\": Value Change" {
      selector: _ -> [_ _ _ _]
      dyn-events: _ -> [_ _ _ _]
      timeout: _ -> [_ _ _ _]
      tunnel: [w1162 w1172 w1223 w1231] -> w1159
      tunnel: "Output" -> [_ w1171 _ _]
      tunnel: [_ _ _ TRUE ("Value (Signaling)")] -> w1157
      tunnel: w1156 -> [w1162 w1170 w1228 w1232]
      tunnel: w1155 -> [w1161 w1169 w1225 w1230]
      tunnel: [w1161 w1168 w1224 w1229] -> w1154
      tunnel: w1153 -> [_ w1167 _ _]
      event Timeout {
        n542 = event-data() -> ()  [unwired: 1 in, 3 out]
      }
      event "Output", "SetCurrent 1 (mA)": Value Change {
        n543 = event-data() -> ()  [unwired: 1 in, 6 out]
        n544 = local read "Initialized?"() -> (w1166:bool)
        n545 = stacked-sequence {
          tunnel: [_ w1190] -> w1163
          frame #0 {
            n546 = Less?(x="SetCurrent 2 (mA)", y="lower limit (mA)") -> (x < y?=w1174:bool)
            n547 = Greater?(x="SetCurrent 2 (mA)", y="upper limit (mA)") -> (0:w1175:bool)
            n548 = Less?(x="SetCurrent 1 (mA)", y="lower limit (mA)") -> (x < y?=w1178:bool)
            n549 = Greater?(x="SetCurrent 1 (mA)", y="upper limit (mA)") -> (0:w1180:bool)
            n550 = case shown="True" w1174 {
              tunnel: "lower limit (mA)" -> [_ w1181]
              frame False {
              }
              frame True {
                n551 = property on="SetCurrent 2 (mA)" class="DigNum (strict)"("Val(Sgnl)"=w1181) -> ()  [unwired: 2 in, 2 out]
              }
            }
            n552 = case shown="True" w1178 {
              tunnel: "lower limit (mA)" -> [_ w1183]
              frame False {
              }
              frame True {
                n553 = property on="SetCurrent 1 (mA)" class="DigNum (strict)"("Val(Sgnl)"=w1183) -> ()  [unwired: 2 in, 2 out]
              }
            }
            n554 = case shown="True" w1175 {
              tunnel: "upper limit (mA)" -> [_ w1182]
              frame False {
              }
              frame True {
                n555 = property on="SetCurrent 2 (mA)" class="DigNum (strict)"("Val(Sgnl)"=w1182) -> ()  [unwired: 2 in, 2 out]
              }
            }
            n556 = case shown="True" w1180 {
              tunnel: "upper limit (mA)" -> [_ w1184]
              frame False {
              }
              frame True {
                n557 = property on="SetCurrent 1 (mA)" class="DigNum (strict)"("Val(Sgnl)"=w1184) -> ()  [unwired: 2 in, 2 out]
              }
            }
          }
          frame #1 {
            w1186 = 1000.0 ("y")
            n558 = local read "SetCurrent 2 (mA)"() -> (w1187:dbl)
            n559 = local read "SetCurrent 1 (mA)"() -> (w1189:dbl)
            n560 = Divide(x=w1189, y=w1186) -> (x/y=w1188:dbl)
            n561 = Divide(x=w1187, y=w1186) -> (x/y=w1185:dbl)
            n562 = Build Array(w1188, w1185) -> (w1190:dbl[])
          }
        }
        n563 = Not Equal?(x=w1166, y=FALSE) -> (x != y?=w1164:bool)
        n564 = case shown="True" w1164 {
          tunnel: [w1192 w1216] -> w1172
          tunnel: w1171 -> [_ w1215]
          tunnel: w1170 -> [w1192 w1214]
          tunnel: w1169 -> [w1191 w1213]
          tunnel: [w1191 w1212] -> w1168
          tunnel: w1167 -> [_ w1208]
          tunnel: w1163 -> [_ w1193]
          frame False {
          }
          frame True {
            w1201 = 1 ("index (col)")
            w1202 = 0 ("disabled index (col)")
            n565 = call-dynamic "6240AData_execute.vi"("6240AData in"=w1214, "SetCurrent (A)"=w1193, "FileFormat"="%3.5f", "Output status"=w1215, "ExecutionIndex"=w1208, "error in (no error)"=w1213) -> ("ActualVoltage (V)"=→"ActualVoltage (V)":dbl[], "ActualCurrent (A)"=w1207:dbl[], "6240AData out"=w1216:refnum<class "6240AData.lvclass">, "appended array"=w1197:timestamp[], "SetCurrentArray"=w1203:dbl[][], "ActualCurrentArray"=w1210:dbl[][], "error out"=w1212:errorcluster)  [unwired: 3 in]
            n566 = property on="ActualCurrent (A)" class="Arr (strict)"("Val(Sgnl)"=w1207) -> ()  [unwired: 2 in, 2 out]
            n567 = Index Array(array=w1210, index (col) #1=w1202, index (col) #2=w1201) -> (element #1=w1211:dbl[], element #2=w1205:dbl[])  [unwired: 2 in]
            n568 = Index Array(array=w1203, index (col) #1=w1202, index (col) #2=w1201) -> (element #1=w1199:dbl[], element #2=w1196:dbl[])  [unwired: 2 in]
            n569 = Bundle("appended array"=w1197, "ActualCurrentArray"=w1211) -> (w1206:T20)  [unwired: 1 in]
            n570 = Bundle("appended array"=w1197, "ActualCurrentArray"=w1205) -> (w1200:T20)  [unwired: 1 in]
            n571 = Bundle("appended array"=w1197, "SetCurrentArray"=w1199) -> (w1198:T21)  [unwired: 1 in]
            n572 = Bundle("appended array"=w1197, "SetCurrentArray"=w1196) -> (w1195:T21)  [unwired: 1 in]
            n573 = Build Array(w1206, w1200, w1198, w1195) -> (→"Graph 6":T22)
          }
        }
      }
      event "Initialize": Value Change {
        n574 = event-data() -> ()  [unwired: 1 in, 6 out]
        n575 = property on="Initialized?" class="Bool (strict)"("Val(Sgnl)"=TRUE ("Value (Signaling)")) -> ()  [unwired: 2 in, 2 out]
        n576 = local read "RUN identifier"() -> (w1217:string)
        n577 = local read "Base Path"() -> (w1218:path)
        n578 = Get Date/Time In Seconds() -> (seconds since 1Jan1904=w1227:timestamp)
        n579 = call-dynamic "6240AData_initialize.vi"("6240AData in"=w1228, "RunName"=w1217, "InstName"="InstName", "start time"=w1227, "base path"=w1218, "VISA"="VISA", "error in (no error)"=w1225, "CtrlLabels"="CtrlLabels", "Voltage limits (V)"="Voltage limits (V)") -> ("6240AData out"=w1223:refnum<class "6240AData.lvclass">, "error out"=w1224:errorcluster)  [unwired: 5 in]
      }
      event "Stop Button": Value Change {
        n580 = event-data() -> ()  [unwired: 1 in, 6 out]
        n581 = call-dynamic "6240AData_terrminate.vi"("error in (no error)"=w1230, "6240AData in"=w1232) -> ("error out"=w1229:errorcluster, "6240AData out"=w1231:refnum<class "6240AData.lvclass">)  [unwired: 8 in]
      }
    }
    "error out (ADCMT6420A)" <- w1154
  }
  n582 = call-dynamic "USBData_terminate.vi"("error in (no error)"=w23, "USBData in"=w24) -> ("error out"=w25:errorcluster)  [unwired: 8 in, 1 out]
  n583 = call-dynamic "LSI336Data_terminate.vi"("error in (no error)"=w13, "LSI336Data in"=w14) -> ("error out"=w12:errorcluster)  [unwired: 8 in, 1 out]
  n584 = call-dynamic "USBData_terminate.vi"("error in (no error)"=w6, "USBData in"=w7) -> ("error out"=w8:errorcluster)  [unwired: 8 in, 1 out]
  n585 = call "LSI218Data_terminate.vi"("error in (no error)"=w17, "LSI218Data in"=w18) -> ("error out"=w16:errorcluster)  [unwired: 8 in, 1 out]
  n586 = local write "error out (USB6210)"(w25) -> ()
  n587 = local write "error out (LSI336)"(w12) -> ()
  n588 = local write "error out (USB6210)"(w8) -> ()
  n589 = local write "error out (LSI218)"(w16) -> ()
